vi "Dresden R2R Sputter 03.02.2018 IY24.vi"() -> ()   [LabVIEW 2009] (continued)
        "CH1_2trns_6" <- w28815
        "CH1_2trns_11" <- w28815
        "CH1_2trns_12" <- w28815
        "CH1_2trns_19" <- w28815
        "CH1_2trns_7" <- w28815
        "CH1_2trns_8" <- w28815
      }
    }
    n23486 = case shown="True" "Clean_trnsfr_2_3" {
      frame #0 {
      }
      frame #1 {
        w28814 = i16? 0
        n23487 = local write "Clean_trnsfr_2_3"(w28814) -> ()
        "CH2_3_trns_0" <- w28814
        "CH2_3_trns_1" <- w28814
        "CH2_3_trns_2" <- w28814
        "CH2_3_trns_4" <- w28814
        "CH2_3_trns_7" <- w28814
        "CH2_3_trns_8" <- w28814
        "CH2_3_trns_12" <- w28814
        "CH2_3_trns_15" <- w28814
        "CH2_3_trns_18" <- w28814
        "CH2_3_trns_19" <- w28814
        "CH2_3_trns_11" <- w28814
        "CH2_3_trns_10" <- w28814
        "CH2_3_trns_3" <- w28814
        "CH2_3_trns_5" <- w28814
        "CH2_3_trns_6" <- w28814
        "CH2_3_trns_9" <- w28814
        "CH2_3_trns_14" <- w28814
        "CH2_3_trns_17" <- w28814
        "CH2_3_trns_16" <- w28814
        "CH2_3_trns_13" <- w28814
        "CH2_3_trns_20" <- w28814
      }
    }
    n23488 = case shown="True" "Clean_trnsfr_3_4" {
      frame #0 {
      }
      frame #1 {
        w28813 = i16? 0
        n23489 = local write "Clean_trnsfr_3_4"(w28813) -> ()
        "CH3_4_trns_0" <- w28813
        "CH3_4_trns_1" <- w28813
        "CH3_4_trns_2" <- w28813
        "CH3_4_trns_4" <- w28813
        "CH3_4_trns_7" <- w28813
        "CH3_4_trns_8" <- w28813
        "CH3_4_trns_12" <- w28813
        "CH3_4_trns_15" <- w28813
        "CH3_4_trns_18" <- w28813
        "CH3_4_trns_19" <- w28813
        "CH3_4_trns_10" <- w28813
        "CH3_4_trns_11" <- w28813
        "CH3_4_trns_3" <- w28813
        "CH3_4_trns_5" <- w28813
        "CH3_4_trns_6" <- w28813
        "CH3_4_trns_9" <- w28813
        "CH3_4_trns_14" <- w28813
        "CH3_4_trns_17" <- w28813
        "CH3_4_trns_16" <- w28813
        "CH3_4_trns_13" <- w28813
        "CH3_4_trns_20" <- w28813
      }
    }
    n23490 = case shown="True" "Clean_trnsfr_2_1" {
      frame #0 {
      }
      frame #1 {
        w28812 = i16? 0
        n23491 = local write "Clean_trnsfr_2_1"(w28812) -> ()
        "CH2_1_trns_0" <- w28812
        "CH2_1_trns_1" <- w28812
        "CH2_1_trns_2" <- w28812
        "CH2_1_trns_3" <- w28812
        "CH2_1_trns_4" <- w28812
        "CH2_1_trns_5" <- w28812
        "CH2_1_trns_7" <- w28812
        "CH2_1_trns_6" <- w28812
        "CH2_1_trns_8" <- w28812
        "CH2_1_trns_9" <- w28812
        "CH2_1_trns_10" <- w28812
        "CH2_1_trns_11" <- w28812
        "CH2_1_trns_12" <- w28812
        "CH2_1_trns_14" <- w28812
        "CH2_1_trns_15" <- w28812
        "CH2_1_trns_17" <- w28812
        "CH2_1_trns_18" <- w28812
        "CH2_1_trns_16" <- w28812
        "CH2_1_trns_19" <- w28812
        "CH2_1_trns_13" <- w28812
        "CH2_1_trns_20" <- w28812
      }
    }
    n23492 = case shown="True" "Clean_trnsfr_3_2" {
      frame #0 {
      }
      frame #1 {
        w28811 = i16? 0
        n23493 = local write "Clean_trnsfr_3_2"(w28811) -> ()
        "CH3_2_trns_0" <- w28811
        "CH3_2_trns_1" <- w28811
        "CH3_2_trns_2" <- w28811
        "CH3_2_trns_3" <- w28811
        "CH3_2_trns_4" <- w28811
        "CH3_2_trns_5" <- w28811
        "CH3_2_trns_7" <- w28811
        "CH3_2_trns_6" <- w28811
        "CH3_2_trns_ 8" <- w28811
        "CH3_2_trns_9" <- w28811
        "CH3_2_trns_10" <- w28811
        "CH3_2_trns_11" <- w28811
        "CH3_2_trns_12" <- w28811
        "CH3_2_trns_14" <- w28811
        "CH3_2_trns_15" <- w28811
        "CH3_2_trns_17" <- w28811
        "CH3_2_trns_18" <- w28811
        "CH3_2_trns_16" <- w28811
        "CH3_2_trns_19" <- w28811
        "CH3_2_trns_13" <- w28811
        "CH3_2_trns_20" <- w28811
      }
    }
    n23494 = case shown="True" "Clean_trnsfr_4_3" {
      frame #0 {
      }
      frame #1 {
        w28810 = i16? 0
        n23495 = local write "Clean_trnsfr_4_3"(w28810) -> ()
        "CH4_3_trns_0" <- w28810
        "CH4_3_trns_1" <- w28810
        "CH4_3_trns_2" <- w28810
        "CH4_3_trns_3" <- w28810
        "CH4_3_trns_5" <- w28810
        "CH4_3_trns_7" <- w28810
        "CH4_3_trns_6" <- w28810
        "CH4_3_trns_8" <- w28810
        "CH4_3_trns_9" <- w28810
        "CH4_3_trns_10" <- w28810
        "CH4_3_trns_4" <- w28810
        "CH4_3_trns_11" <- w28810
        "CH4_3_trns_14" <- w28810
        "CH4_3_trns_15" <- w28810
        "CH4_3_trns_17" <- w28810
        "CH4_3_trns_18" <- w28810
        "CH4_3_trns_19" <- w28810
        "CH4_3_trns_16" <- w28810
        "CH4_3_trns_13" <- w28810
        "CH4_3_trns_20" <- w28810
      }
    }
    n23496 = case shown="True" "Routine_check" {
      frame #0 {
      }
      frame #1 {
        w28807 = i16? 0
        n23497 = local write "Routine_check"(w28807) -> ()
        "RC_1" <- w28807
        "RC_2" <- w28807
        "RC_3" <- w28807
        "RC_4" <- w28807
        "RC_5" <- w28807
        "RC_6" <- w28807
        "RC_7" <- w28807
        "RC_8" <- w28807
        "RC_9" <- w28807
        "RC_10" <- w28807
        "RC_11" <- w28807
        "RC_12" <- w28807
        "RC_13" <- w28807
      }
    }
    n23498 = stacked-sequence {
      frame #0 {
        # "MAIN TRANSFER CLEAN"
        n23499 = case shown="True" "Clean_main_trns" {
          frame #0 {
          }
          frame #1 {
            w28809 = i16? 0 ("a1")
            n23500 = local write "Clean_main_trns"(w28809) -> ()
            "MT4" <- w28809
            "MT1" <- w28809
            "MT5" <- w28809
            "MT6" <- w28809
            "MT3" <- w28809
            "MT2" <- w28809
            "MT7" <- w28809
            "MT13" <- w28809
            "MT9" <- w28809
            "MT11" <- w28809
            "MT8" <- w28809
            "MT10" <- w28809
            "MT12" <- w28809
            "MT14" <- w28809
            "MT15" <- w28809
            "MT18" <- w28809
            "MT16" <- w28809
            "MT17" <- w28809
            "MT19" <- w28809
            "MT20" <- w28809
            "MTF" <- w28809
          }
        }
      }
    }
    n23501 = case shown="True" "Clean_MW_Coating" {
      frame #0 {
      }
      frame #1 {
        w28806 = i16? 0 ("a1")
        n23502 = local write "Clean_MW_Coating"(w28806) -> ()
        "SMW1" <- w28806
        "SMW2" <- w28806
        "SMW4" <- w28806
        "SMW5" <- w28806
        "SMW6" <- w28806
        "SMW9" <- w28806
        "SMW8" <- w28806
        "SMW11" <- w28806
        "SMW12" <- w28806
        "SMW13" <- w28806
        "SMW14" <- w28806
        "SMW15" <- w28806
        "SMW3" <- w28806
        "SMW16" <- w28806
        "SMW17" <- w28806
        "SMW18" <- w28806
        "SMW19" <- w28806
        "SMW21" <- w28806
        "SMW22" <- w28806
        "SMW23" <- w28806
        "SMW26" <- w28806
        "SMW7" <- w28806
        "SMW10" <- w28806
        "SMW20" <- w28806
        "SMW18b" <- w28806
        "SMW24" <- w28806
        "SMW25" <- w28806
        "SMW1 2" <- w28806
      }
    }
    n23503 = case shown="True" "Clean_Single_DC1" {
      frame #0 {
      }
      frame #1 {
        w28805 = i16? 0 ("a1")
        n23504 = local write "Clean_Single_DC1"(w28805) -> ()
        "SDC1 1" <- w28805
        "SDC1 2" <- w28805
        "SDC1 3" <- w28805
        "SDC1 4" <- w28805
        "SDC1 5" <- w28805
        "SDC1 6" <- w28805
        "SDC1 7" <- w28805
        "SDC1 8" <- w28805
        "SDC1 9" <- w28805
        "SDC1 10" <- w28805
        "SDC1 11" <- w28805
        "SDC1 13" <- w28805
        "SDC1 14" <- w28805
        "SDC1 17" <- w28805
        "SDC1 18" <- w28805
        "SDC1 20" <- w28805
        "SDC1 21" <- w28805
        "SDC1 22" <- w28805
        "SDC1 23" <- w28805
        "SDC1 24" <- w28805
        "SDC1 25" <- w28805
        "SDC1 26" <- w28805
        "SDC1 27" <- w28805
        "SDC1 28" <- w28805
        "SDC1 29" <- w28805
        "SDC1 30" <- w28805
        "SDC1 21b" <- w28805
        "SDC1 2b" <- w28805
        "SDC1 7b" <- w28805
        "SDC1 10b" <- w28805
        "SDC1 13b" <- w28805
        "SDC1 14b" <- w28805
        "SDC1 27b" <- w28805
        "SDC1 27c" <- w28805
        "SDC1 12" <- w28805
      }
    }
    n23505 = case shown="True" "Clean_Single_DC2" {
      frame #0 {
      }
      frame #1 {
        w28804 = i16? 0 ("a1")
        n23506 = local write "Clean_Single_DC2"(w28804) -> ()
        "SDC2 1" <- w28804
        "SDC2 2" <- w28804
        "SDC2 4" <- w28804
        "SDC2 3" <- w28804
        "SDC2 5" <- w28804
        "SDC2 6" <- w28804
        "SDC2 7" <- w28804
        "SDC2 8" <- w28804
        "SDC2 9" <- w28804
        "SDC2 10" <- w28804
        "SDC2 11" <- w28804
        "SDC2 12" <- w28804
        "SDC2 13" <- w28804
        "SDC2 14" <- w28804
        "SDC2 17" <- w28804
        "SDC2 18" <- w28804
        "SDC2 20" <- w28804
        "SDC2 21" <- w28804
        "SDC2 22" <- w28804
        "SDC2 23" <- w28804
        "SDC2 24" <- w28804
        "SDC2 25" <- w28804
        "SDC2 26" <- w28804
        "SDC2 27" <- w28804
        "SDC2 28" <- w28804
        "SDC2 29" <- w28804
        "SDC2 30" <- w28804
        "SDC2 21b" <- w28804
        "SDC2 3b" <- w28804
        "SDC2 b" <- w28804
        "SDC2 10b" <- w28804
        "SDC2 15" <- w28804
        "SDC2 16" <- w28804
        "SDC2 28b" <- w28804
        "SDC2 28c" <- w28804
        "SDC2 19" <- w28804
      }
    }
    n23507 = case shown="True" "Clean_Single_RF" {
      frame #0 {
      }
      frame #1 {
        w28803 = i16? 0 ("a1")
        n23508 = local write "Clean_Single_RF"(w28803) -> ()
        "SRF 1" <- w28803
        "SRF 2" <- w28803
        "SRF 3" <- w28803
        "SRF 4" <- w28803
        "SRF 5" <- w28803
        "SRF 6" <- w28803
        "SRF 7" <- w28803
        "SRF 8" <- w28803
        "SRF 9" <- w28803
        "SRF 10" <- w28803
        "SRF 11" <- w28803
        "SRF 12" <- w28803
        "SRF 13" <- w28803
        "SRF 14" <- w28803
        "SRF 17" <- w28803
        "SRF 18" <- w28803
        "SRF 19" <- w28803
        "SRF 20" <- w28803
        "SRF 21" <- w28803
        "SRF 22" <- w28803
        "SRF 23" <- w28803
        "SRF 24" <- w28803
        "SRF 25" <- w28803
        "SRF 26" <- w28803
        "SRF 27" <- w28803
        "SRF 28" <- w28803
        "SRF 29" <- w28803
        "SRF 30" <- w28803
        "SRF 21b" <- w28803
        "SRF 4b" <- w28803
        "SRF 7b" <- w28803
        "SRF 8b" <- w28803
        "SRF 27b" <- w28803
        "SRF 27c" <- w28803
        "SRF 15" <- w28803
      }
    }
    n23509 = case shown="True" "Clean_Combo" {
      frame #0 {
      }
      frame #1 {
        w28802 = i16? 0 ("a1")
        n23510 = local write "Clean_Combo"(w28802) -> ()
        "SCMB1" <- w28802
        "SCMB2" <- w28802
        "SCMB3" <- w28802
        "SCMB4" <- w28802
        "SCMB5" <- w28802
        "SCMB6" <- w28802
        "SCMB7" <- w28802
        "SCMB8" <- w28802
        "SCMB9" <- w28802
        "SCMB10" <- w28802
        "SCMB11" <- w28802
        "SCMB12" <- w28802
        "SCMB13" <- w28802
        "SCMB14" <- w28802
        "SCMB15" <- w28802
        "SCMB16" <- w28802
        "SCMB17" <- w28802
        "SCMB18" <- w28802
        "SCMB19" <- w28802
        "SCMB20" <- w28802
        "SCMB21" <- w28802
        "SCMB22" <- w28802
        "SCMB23" <- w28802
        "SCMB24" <- w28802
        "SCMB25" <- w28802
        "SCMB26" <- w28802
        "SCMB27" <- w28802
        "SCMB28" <- w28802
        "SCMB29" <- w28802
        "SCMB30" <- w28802
        "SCMB31" <- w28802
        "SCMB32" <- w28802
        "SCMB33" <- w28802
        "SCMB34" <- w28802
        "SCMB35" <- w28802
        "SCMB36" <- w28802
        "SCMB37" <- w28802
        "SCMB38" <- w28802
        "SCMB39" <- w28802
        "SCMB40" <- w28802
        "SCMB41" <- w28802
        "SCMB42" <- w28802
        "SCMB43" <- w28802
        "SCMB44" <- w28802
        "SCMB45" <- w28802
        "SCMB46" <- w28802
        "SCMB47" <- w28802
        "SCMB48" <- w28802
        "SCMB49" <- w28802
        "SCMB50" <- w28802
        "SCMB51" <- w28802
        "SCMB52" <- w28802
        "SCMB53" <- w28802
        "SCMB54" <- w28802
        "SCMB55" <- w28802
        "SCMB56" <- w28802
        "SCMB57" <- w28802
        "SCMB58" <- w28802
        "SCMB59" <- w28802
        "SCMB60" <- w28802
        "SCMB61" <- w28802
        "SCMB62" <- w28802
        "SCMB63" <- w28802
        "SCMB64" <- w28802
        "SCMB65" <- w28802
        "SCMB66" <- w28802
        "SCMB67" <- w28802
        "SCMB68" <- w28802
        "SCMB69" <- w28802
        "SCMB70" <- w28802
        "SCMB71" <- w28802
        "SCMB72" <- w28802
        "SCMB73" <- w28802
        "SCMB74" <- w28802
        "SCMB75" <- w28802
        "SCMB0" <- w28802
        "SCMB0 2" <- w28802
      }
    }
  }
  n23511 = VISA Close(VISA resource name=w809, error in (no error)=w733) -> ()  [unwired: 1 out]
  n23512 = while {
    stop <- FALSE stop-if-true
    n23513 = local read "Path"() -> (w28838:string)
    n23514 = Wait Until Next ms Multiple(millisecond multiple=u32 300) -> ()  [unwired: 1 out]
    n23515 = String To Path(string=w28838) -> (path=w28839:path)
    n23516 = Not Equal?(x=w28838, y="") -> (x != y?=w28840:bool)
    n23517 = case shown="True" w28840 {
      tunnel: w28839 -> [_ w28936]
      frame #0 {
      }
      frame #1 {
        # "Thickness Monitor AC/DEAC\nMaterial Density\nZ factor\nTooling Factor"
        # "Target Material\nIgnition Power\nTarget clean Power AC/DEAC\nTarget clean Power\nTarget clean Time\nTarget Material\nIgnition Power\nTarget clean Power AC/DEAC\nTarget clean Power\nTarget clean Time\nRegion1 active/deactive\nch2-Coating Power\nch3-Coating Power\nRegion2 active/deactive\nch2-Coating Power\nch3-Coating Power\nRegion3 active/deactive\nch2-Coating Power\nch3-Coating Power\nRegion4 active/deactive\nch2-Coating Power\nch3-Coating Power\nRegion5 active/deactive\nch2-Coating Power\nch3-Coating Power\nInterval Length"
        # "Target Material\nRamp Up Time Active/deactive\nRamp Up Time\nIgnition Power\nTarget Clean  ACT/DEACT\nTarget Clean Power\nTarget Clean Time\nRegion1 active/deactive\nCoating Power\nInterval Length\nRegion2 active/deactive\nCoating Powe\nRegion3 active/deactive\nCoating Power\nRegion4 active/deactive\nCoating Power\nRegion5 active/deactive\nCoating Power\nRamp DownTime activedeactive\nRamp Down Time"
        # "Recipe Selection"
        # "Ar Flow\nSet Pressure"
        # "DC SELECTION\nTarget Material\nIgnition Power\nTarget Clean  ACT/DEACT\nTarget Clean Power\nTarget Clean Time\nRegion1 active/deactive\nCoating Power\nInterval Length\nRegion2 active/deactive\nCoating Powe\nRegion3 active/deactive\nCoating Power\nRegion4 active/deactive\nCoating Power\nRegion5 active/deactive\nCoating Power"
        # "Microwave Plasma Power\n\nMicrowave Duration\nMicrowave Times"
        # "Coating Selection"
        # "Thickness Selection\nTarget Thickness Value\nTime"
        # "Min. Diameter\nMax. Diameter\nWeb Thickness\nWeb Speed\nTension  Value\nTotal Length"
        # "Web Selection"
        # "Substrate Material"
        # "Recipe Name"
        n23518 = call-poly <vilib>:"Read From Spreadsheet File.vi"("file path (dialog if empty)"=w28936) -> ("all rows"=w29282:string[][])  [unwired: 6 in, 4 out]
        n23519 = Index Array(array=w29282, index (row) #1=1 ("disabled index (row)"), index (col) #1=3 ("disabled index (col)"), index (row) #2=4 ("disabled index (row)"), index (col) #2=2 ("disabled index (col)"), index (row) #3=7 ("disabled index (row)"), index (col) #3=2 ("disabled index (col)"), index (row) #4=9 ("disabled index (row)"), index (col) #4=3 ("disabled index (col)"), index (row) #5=12 ("disabled index (row)"), index (col) #5=2 ("disabled index (col)"), index (row) #6=13 ("disabled index (row)"), index (col) #6=2 ("disabled index (col)"), index (row) #7=14 ("disabled index (row)"), index (col) #7=2 ("disabled index (col)"), index (row) #8=15 ("disabled index (row)"), index (col) #8=2 ("disabled index (col)"), index (row) #9=16 ("disabled index (row)"), index (col) #9=2 ("disabled index (col)"), index (row) #10=17 ("disabled index (row)"), index (col) #10=3 ("disabled index (col)"), index (row) #11=20 ("disabled index (row)"), index (col) #11=2 ("disabled index (col)"), index (row) #12=21 ("disabled index (row)"), index (col) #12=3 ("disabled index (col)"), index (row) #13=22 ("disabled index (row)"), index (col) #13=3 ("disabled index (col)"), index (row) #14=25 ("disabled index (row)"), index (col) #14=2 ("disabled index (col)"), index (row) #15=27 ("disabled index (row)"), index (col) #15=1 ("disabled index (col)"), index (row) #16=28 ("disabled index (row)"), index (col) #16=1 ("disabled index (col)"), index (row) #17=29 ("disabled index (row)"), index (col) #17=4 ("disabled index (col)"), index (row) #18=34 ("disabled index (row)"), index (col) #18=2 ("disabled index (col)"), index (row) #19=35 ("disabled index (row)"), index (col) #19=2 ("disabled index (col)"), index (row) #20=36 ("disabled index (row)"), index (col) #20=2 ("disabled index (col)"), index (row) #21=37 ("disabled index (row)"), index (col) #21=2 ("disabled index (col)"), index (row) #22=38 ("disabled index (row)"), index (col) #22=2 ("disabled index (col)"), index (row) #23=39 ("disabled index (row)"), index (col) #23=2 ("disabled index (col)"), index (row) #24=40 ("disabled index (row)"), index (col) #24=3 ("disabled index (col)"), index (row) #25=41 ("disabled index (row)"), index (col) #25=2 ("disabled index (col)"), index (row) #26=42 ("disabled index (row)"), index (col) #26=2 ("disabled index (col)"), index (row) #27=43 ("disabled index (row)"), index (col) #27=3 ("disabled index (col)"), index (row) #28=44 ("disabled index (row)"), index (col) #28=2 ("disabled index (col)"), index (row) #29=45 ("disabled index (row)"), index (col) #29=3 ("disabled index (col)"), index (row) #30=46 ("disabled index (row)"), index (col) #30=2 ("disabled index (col)"), index (row) #31=47 ("disabled index (row)"), index (col) #31=3 ("disabled index (col)"), index (row) #32=48 ("disabled index (row)"), index (col) #32=2 ("disabled index (col)"), index (row) #33=49 ("disabled index (row)"), index (col) #33=3 ("disabled index (col)"), index (row) #34=50 ("disabled index (row)"), index (col) #34=2 ("disabled index (col)"), index (row) #35=53 ("disabled index (row)"), index (col) #35=2 ("disabled index (col)"), index (row) #36=54 ("disabled index (row)"), index (col) #36=2 ("disabled index (col)"), index (row) #37=55 ("disabled index (row)"), index (col) #37=2 ("disabled index (col)"), index (row) #38=56 ("disabled index (row)"), index (col) #38=2 ("disabled index (col)"), index (row) #39=57 ("disabled index (row)"), index (col) #39=2 ("index (col)"), index (row) #40=58 ("disabled index (row)"), index (col) #40=2 ("index (col)"), index (row) #41=59 ("disabled index (row)"), index (col) #41=2 ("index (col)"), index (row) #42=60 ("disabled index (row)"), index (col) #42=3 ("index (col)"), index (row) #43=61 ("disabled index (row)"), index (col) #43=2 ("index (col)"), index (row) #44=62 ("disabled index (row)"), index (col) #44=2 ("index (col)"), index (row) #45=63 ("disabled index (row)"), index (col) #45=3 ("index (col)"), index (row) #46=64 ("disabled index (row)"), index (col) #46=2 ("index (col)"), index (row) #47=65 ("disabled index (row)"), index (col) #47=3 ("disabled index (row)"), index (row) #48=66 ("disabled index (row)"), index (col) #48=2 ("disabled index (col)"), index (row) #49=67 ("disabled index (row)"), index (col) #49=3 ("index (col)"), index (row) #50=68 ("disabled index (row)"), index (col) #50=2 ("index (col)"), index (row) #51=69 ("disabled index (row)"), index (col) #51=3 ("index (col)"), index (row) #52=70 ("disabled index (row)"), index (col) #52=2 ("index (col)"), index (row) #53=71 ("disabled index (row)"), index (col) #53=2 ("disabled index (col)"), index (row) #54=72 ("disabled index (row)"), index (col) #54=3 ("index (col)"), index (row) #55=78 ("disabled index (row)"), index (col) #55=2 ("index (col)"), index (row) #56=79 ("disabled index (row)"), index (col) #56=2 ("index (col)"), index (row) #57=80 ("disabled index (row)"), index (col) #57=2 ("index (col)"), index (row) #58=81 ("disabled index (row)"), index (col) #58=2 ("index (col)"), index (row) #59=82 ("disabled index (row)"), index (col) #59=2 ("index (col)"), index (row) #60=83 ("disabled index (row)"), index (col) #60=2 ("index (col)"), index (row) #61=84 ("disabled index (row)"), index (col) #61=2 ("index (col)"), index (row) #62=85 ("disabled index (row)"), index (col) #62=2 ("index (col)"), index (row) #63=86 ("disabled index (row)"), index (col) #63=2 ("index (col)"), index (row) #64=87 ("disabled index (row)"), index (col) #64=2 ("index (col)"), index (row) #65=88 ("disabled index (row)"), index (col) #65=3 ("index (col)"), index (row) #66=89 ("disabled index (row)"), index (col) #66=2 ("index (col)"), index (row) #67=90 ("disabled index (row)"), index (col) #67=2 ("index (col)"), index (row) #68=91 ("disabled index (row)"), index (col) #68=3 ("index (col)"), index (row) #69=92 ("disabled index (row)"), index (col) #69=2 ("index (col)"), index (row) #70=93 ("disabled index (row)"), index (col) #70=2 ("index (col)"), index (row) #71=94 ("disabled index (row)"), index (col) #71=3 ("index (col)"), index (row) #72=95 ("disabled index (row)"), index (col) #72=2 ("disabled index (col)"), index (row) #73=96 ("disabled index (row)"), index (col) #73=2 ("index (col)"), index (row) #74=97 ("disabled index (row)"), index (col) #74=3 ("index (col)"), index (row) #75=98 ("disabled index (row)"), index (col) #75=2 ("index (col)"), index (row) #76=99 ("disabled index (row)"), index (col) #76=2 ("index (col)"), index (row) #77=100 ("disabled index (row)"), index (col) #77=3 ("index (col)"), index (row) #78=101 ("disabled index (row)"), index (col) #78=2 ("index (col)"), index (row) #79=102 ("disabled index (row)"), index (col) #79=2 ("index (col)"), index (row) #80=103 ("disabled index (row)"), index (col) #80=2 ("index (col)"), index (row) #81=104 ("disabled index (row)"), index (col) #81=2 ("disabled index (row)"), index (row) #82=108 ("disabled index (row)"), index (col) #82=2 ("index (col)"), index (row) #83=109 ("disabled index (row)"), index (col) #83=2 ("index (col)"), index (row) #84=113 ("disabled index (row)"), index (col) #84=2 ("index (col)"), index (row) #85=114 ("disabled index (row)"), index (col) #85=3 ("index (col)"), index (row) #86=115 ("disabled index (row)"), index (col) #86=2 ("index (col)"), index (row) #87=116 ("disabled index (row)"), index (col) #87=2 ("index (col)")) -> (element #1=w29273:string, element #2=w29269:string, element #3=w29268:string, element #4=w29266:string, element #5=w29257:string, element #6=w29256:string, element #7=w29255:string, element #8=w29252:string, element #9=w29249:string, element #10=w29248:string, element #11=w29247:string, element #12=w29242:string, element #13=w29241:string, element #14=w29239:string, element #15=w29236:string, element #16=w28926:string, element #17=w28925:string, element #18=w28924:string, element #19=w29185:string, element #20=w29184:string, element #21=w29183:string, element #22=w29182:string, element #23=w29181:string, element #24=w29180:string, element #25=w29179:string, element #26=w29178:string, element #27=w29177:string, element #28=w29176:string, element #29=w29175:string, element #30=w29174:string, element #31=w29173:string, element #32=w29172:string, element #33=w29171:string, element #34=w29168:string, element #35=w29133:string, element #36=w29130:string, element #37=w29128:string, element #38=w29097:string, element #39=w29096:string, element #40=w29095:string, element #41=w29094:string, element #42=w29093:string, element #43=w29092:string, element #44=w29091:string, element #45=w29090:string, element #46=w29089:string, element #47=w29088:string, element #48=w29087:string, element #49=w29086:string, element #50=w29085:string, element #51=w29084:string, element #52=w29083:string, element #53=w29082:string, element #54=w29081:string, element #55=w29021:string, element #56=w29020:string, element #57=w29019:string, element #58=w28998:string, element #59=w28997:string, element #60=w28996:string, element #61=w28995:string, element #62=w28994:string, element #63=w28992:string, element #64=w28979:string, element #65=w28978:string, element #66=w28977:string, element #67=w28976:string, element #68=w28971:string, element #69=w28970:string, element #70=w28969:string, element #71=w28968:string, element #72=w28965:string, element #73=w28964:string, element #74=w28963:string, element #75=w28962:string, element #76=w28959:string, element #77=w28958:string, element #78=w28956:string, element #79=w28955:string, element #80=w28954:string, element #81=w28913:string, element #82=w28912:string, element #83=w28906:string, element #84=w28904:string, element #85=w28903:string, element #86=w28902:string, element #87=w28901:string)
        n23520 = Equal?(x="Active", y=w28904) -> (x = y?=w28905:bool)
        n23521 = case shown="True" w28905 {
          frame #0 {
            n23522 = local write "Thickness_Monitor_Active"(FALSE ("Thickness_Monitor_Active")) -> ()
          }
          frame #1 {
            n23523 = local write "Thickness_Monitor_Active"(TRUE ("Thickness_Monitor_Active")) -> ()
          }
        }
        n23524 = Scan Value(string=w28913, format string="") -> (value=w28915:dbl)  [unwired: 1 in, 1 out]
        n23525 = Scan Value(string=w28912, format string="") -> (value=w28950:dbl)  [unwired: 1 in, 1 out]
        n23526 = Scan Value(string=w28906, format string="") -> (value=w28947:dbl)  [unwired: 1 in, 1 out]
        n23527 = Scan Value(string=w28903, format string="") -> (value=w28945:dbl)  [unwired: 1 in, 1 out]
        n23528 = Scan Value(string=w28902, format string="") -> (value=w28942:dbl)  [unwired: 1 in, 1 out]
        n23529 = Scan Value(string=w28901, format string="") -> (value=w28941:dbl)  [unwired: 1 in, 1 out]
        n23530 = local write "R Material_density"(w28945) -> ()
        n23531 = local write "R Z_factor"(w28942) -> ()
        n23532 = local write "R Toooling_factor"(w28941) -> ()
        n23533 = local write "R Cmb Number of pairs"(w28915) -> ()
        n23534 = local write "R Argon Flow sccm"(w28950) -> ()
        n23535 = local write "R Set Pressure mtorr"(w28947) -> ()
        n23536 = local write "Recipe Name"(w29273) -> ()
        n23537 = local write "Substrate Material"(w29269) -> ()
        n23538 = local write "R Cmb Ch3 Target material"(w28996) -> ()
        n23539 = local write "R Cmb Ch2 Target material"(w29021) -> ()
        n23540 = Scan Value(string=w28998, format string="") -> (value=w29016:dbl)  [unwired: 1 in, 1 out]
        n23541 = Scan Value(string=w29020, format string="") -> (value=w29024:dbl)  [unwired: 1 in, 1 out]
        n23542 = Scan Value(string=w28997, format string="") -> (value=w29015:dbl)  [unwired: 1 in, 1 out]
        n23543 = Scan Value(string=w28995, format string="") -> (value=w29013:dbl)  [unwired: 1 in, 1 out]
        n23544 = Scan Value(string=w28979, format string="") -> (value=w29009:dbl)  [unwired: 1 in, 1 out]
        n23545 = Scan Value(string=w28992, format string="") -> (value=w29010:dbl)  [unwired: 1 in, 1 out]
        n23546 = Scan Value(string=w28970, format string="") -> (value=w28973:dbl)  [unwired: 1 in, 1 out]
        n23547 = Scan Value(string=w28964, format string="") -> (value=w28966:dbl)  [unwired: 1 in, 1 out]
        n23548 = Scan Value(string=w28969, format string="") -> (value=w28972:dbl)  [unwired: 1 in, 1 out]
        n23549 = Scan Value(string=w28955, format string="") -> (value=w28953:dbl)  [unwired: 1 in, 1 out]
        n23550 = Scan Value(string=w28976, format string="") -> (value=w28974:dbl)  [unwired: 1 in, 1 out]
        n23551 = Scan Value(string=w28965, format string="") -> (value=w28967:dbl)  [unwired: 1 in, 1 out]
        n23552 = Scan Value(string=w28977, format string="") -> (value=w28975:dbl)  [unwired: 1 in, 1 out]
        n23553 = Scan Value(string=w28956, format string="") -> (value=w28957:dbl)  [unwired: 1 in, 1 out]
        n23554 = Scan Value(string=w28954, format string="") -> (value=w28952:dbl)  [unwired: 1 in, 1 out]
        n23555 = local write "R Cmb Ch2 DC Ignition Power"(w29024) -> ()
        n23556 = Scan Value(string=w28962, format string="") -> (value=w28961:dbl)  [unwired: 1 in, 1 out]
        n23557 = Scan Value(string=w28959, format string="") -> (value=w28960:dbl)  [unwired: 1 in, 1 out]
        n23558 = local write "R Cmb Ch2 DC Target Clean Power"(w29016) -> ()
        n23559 = local write "R Cmb Ch2 DC Target Clean Time"(w29015) -> ()
        n23560 = Equal?(x="Active", y=w28971) -> (x = y?=w29005:bool)
        n23561 = Equal?(x="Active", y=w28978) -> (x = y?=w29007:bool)
        n23562 = local write "R Cmb Ch3 DC Ignition Power"(w29013) -> ()
        n23563 = local write "R Cmb Ch3 DC Target Clean Power"(w29010) -> ()
        n23564 = local write "R Cmb Ch3 DC Target Clean Time"(w29009) -> ()
        n23565 = Equal?(x="Active", y=w28968) -> (x = y?=w29003:bool)
        n23566 = Equal?(x="Active", y=w29019) -> (x = y?=w29022:bool)
        n23567 = Equal?(x="Active", y=w28994) -> (x = y?=w29011:bool)
        n23568 = local write "R Cmb Ch2 Step1 Coating Power"(w28975) -> ()
        n23569 = local write "R Cmb Ch3 Step1 Coating Power"(w28974) -> ()
        n23570 = Equal?(x="Active", y=w28963) -> (x = y?=w29000:bool)
        n23571 = case shown="False" w29005 {
          frame #0 {
            n23572 = local write "R Cmb Ch2 Step2 Coating Power Active"(FALSE ("R Cmb Ch2 Step2 Coating Power Active")) -> ()
          }
          frame #1 {
            n23573 = local write "R Cmb Ch2 Step2 Coating Power Active"(TRUE ("R Cmb Ch2 Step2 Coating Power Active")) -> ()
          }
        }
        n23574 = local write "R Cmb Ch3 Step5 Coating Power"(w28953) -> ()
        n23575 = Equal?(x="Single", y=w29268) -> (x = y?=w29279:bool)
        n23576 = case shown="False" w29007 {
          frame #0 {
            n23577 = local write "R Cmb Ch2 Step1 Coating Power Active"(FALSE ("R Cmb Ch2 Step1 Coating Power Active")) -> ()
          }
          frame #1 {
            n23578 = local write "R Cmb Ch2 Step1 Coating Power Active"(TRUE ("R Cmb Ch2 Step1 Coating Power Active")) -> ()
          }
        }
        n23579 = case shown="False" w29022 {
          frame #0 {
            n23580 = local write "R Cmb Ch2 DC Target Clean Power Active"(FALSE ("R Cmb Ch2 DC Target Clean Power Active")) -> ()
          }
          frame #1 {
            n23581 = local write "R Cmb Ch2 DC Target Clean Power Active"(TRUE ("R Cmb Ch2 DC Target Clean Power Active")) -> ()
          }
        }
        n23582 = case shown="False" w29003 {
          frame #0 {
            n23583 = local write "R Cmb Ch2 Step3 Coating Power Active"(FALSE ("R Cmb Ch2 Step3 Coating Power Active")) -> ()
          }
          frame #1 {
            n23584 = local write "R Cmb Ch2 Step3 Coating Power Active"(TRUE ("R Cmb Ch2 Step3 Coating Power Active")) -> ()
          }
        }
        n23585 = Equal?(x="Active", y=w28958) -> (x = y?=w28999:bool)
        n23586 = local write "R Cmb Interval length"(w28952) -> ()
        n23587 = Equal?(x="Web", y=w29266) -> (x = y?=w29350:bool)
        n23588 = local write "R Cmb Ch2 Step5 Coating Power"(w28957) -> ()
        n23589 = case shown="False" w29011 {
          frame #0 {
            n23590 = local write "R Cmb Ch3 DC Target Clean Power Active"(FALSE ("R Cmb Ch3 DC Target Clean Power Active")) -> ()
          }
          frame #1 {
            n23591 = local write "R Cmb Ch3 DC Target Clean Power Active"(TRUE ("R Cmb Ch3 DC Target Clean Power Active")) -> ()
          }
        }
        n23592 = local write "R Cmb Ch2 Step3 Coating Power"(w28967) -> ()
        n23593 = local write "R Cmb Ch2 Step4 Coating Power"(w28961) -> ()
        n23594 = local write "R Cmb Ch3 Step3 Coating Power"(w28966) -> ()
        n23595 = local write "R Cmb Ch3 Step4 Coating Power"(w28960) -> ()
        n23596 = case shown="True" w29000 {
          frame #0 {
            n23597 = local write "R Cmb Ch2 Step4 Coating Power Active"(FALSE ("R Cmb Ch2 Step4 Coating Power Active")) -> ()
          }
          frame #1 {
            n23598 = local write "R Cmb Ch2 Step4 Coating Power Active"(TRUE ("R Cmb Ch2 Step4 Coating Power Active")) -> ()
          }
        }
        n23599 = Equal?(x="Combination", y=w29268) -> (x = y?=w29280:bool)
        n23600 = local write "R Cmb Ch2 Step2 Coating Power"(w28973) -> ()
        n23601 = local write "R Cmb Ch3 Step2 Coating Power"(w28972) -> ()
        n23602 = Equal?(x="Other", y=w29266) -> (x = y?=w29349:bool)
        n23603 = case shown="True" w28999 {
          frame #0 {
            n23604 = local write "R Cmb Ch2 Step5 Coating Power Active"(FALSE ("R Cmb Ch2 Step5 Coating Power Active")) -> ()
          }
          frame #1 {
            n23605 = local write "R Cmb Ch2 Step5 Coating Power Active"(TRUE ("R Cmb Ch2 Step5 Coating Power Active")) -> ()
          }
        }
        n23606 = local write "R Single DC Target material"(w29185) -> ()
        n23607 = Equal?(x="DC Sputter", y=w29239) -> (x = y?=w29291:bool)
        n23608 = Equal?(x="Microwave Plasma", y=w29239) -> (x = y?=w29292:bool)
        n23609 = Equal?(x="RF Sputter", y=w29239) -> (x = y?=w29287:bool)
        n23610 = Equal?(x="Thickness", y=w29247) -> (x = y?=w29306:bool)
        n23611 = Build Array(FALSE, w29279, w29280) -> (w29275:bool[])
        n23612 = Equal?(x="Active", y=w29183) -> (x = y?=w29212:bool)
        n23613 = Equal?(x="Active", y=w29180) -> (x = y?=w29207:bool)
        n23614 = Build Array(FALSE, w29350, w29349) -> (w29354:bool[])
        n23615 = Equal?(x="Time", y=w29247) -> (x = y?=w29307:bool)
        n23616 = Equal?(x="Active", y=w29177) -> (x = y?=w29206:bool)
        n23617 = Scan Value(string=w29184, format string="") -> (value=w29214:dbl)  [unwired: 1 in, 1 out]
        n23618 = Equal?(x="Active", y=w29175) -> (x = y?=w29203:bool)
        n23619 = local write "R Single RF Target material"(w29133) -> ()
        n23620 = Boolean Array To Number(Boolean array=w29275) -> (number=w29276:u32)
        n23621 = Equal?(x="Active", y=w29173) -> (x = y?=w29202:bool)
        n23622 = Equal?(x="Active", y=w29171) -> (x = y?=w29187:bool)
        n23623 = case shown="True" w29212 {
          frame #0 {
            n23624 = local write "R Single DC Target Clean"(FALSE ("R Single DC Target Clean")) -> ()
          }
          frame #1 {
            n23625 = local write "R Single DC Target Clean"(TRUE ("R Single DC Target Clean")) -> ()
          }
        }
        n23626 = Boolean Array To Number(Boolean array=w29354) -> (number=w29353:u32)
        n23627 = case shown="True" w29207 {
          frame #0 {
            n23628 = local write "R Single DC Step1 Coating Power Active"(FALSE ("R Single DC Step1 Coating Power Active")) -> ()
          }
          frame #1 {
            n23629 = local write "R Single DC Step1 Coating Power Active"(TRUE ("R Single DC Step1 Coating Power Active")) -> ()
          }
        }
        n23630 = Scan Value(string=w29182, format string="") -> (value=w29196:dbl)  [unwired: 1 in, 1 out]
        n23631 = Scan Value(string=w29181, format string="") -> (value=w29195:dbl)  [unwired: 1 in, 1 out]
        n23632 = Equal?(x="Active", y=w29130) -> (x = y?=w29166:bool)
        n23633 = Scan Value(string=w29179, format string="") -> (value=w29210:dbl)  [unwired: 1 in, 1 out]
        n23634 = Mantissa & Exponent(0:w29276) -> (2:w29281:dbl)  [unwired: 1 out]
        n23635 = Equal?(x="Active", y=w29093) -> (x = y?=w29163:bool)
        n23636 = Equal?(x="Active", y=w29096) -> (x = y?=w29199:bool)
        n23637 = Equal?(x="Active", y=w29090) -> (x = y?=w29160:bool)
        n23638 = Equal?(x="Active", y=w29088) -> (x = y?=w29159:bool)
        n23639 = Scan Value(string=w29178, format string="") -> (value=w29194:dbl)  [unwired: 1 in, 1 out]
        n23640 = Equal?(x="Active", y=w29086) -> (x = y?=w29156:bool)
        n23641 = case shown="False" w29206 {
          frame #0 {
            n23642 = local write "R Single DC Step2 Coating Power Active"(FALSE ("R Single DC Step2 Coating Power Active")) -> ()
          }
          frame #1 {
            n23643 = local write "R Single DC Step2 Coating Power Active"(TRUE ("R Single DC Step2 Coating Power Active")) -> ()
          }
        }
        n23644 = local write "R Single DC Ignition Power"(w29214) -> ()
        n23645 = case shown="False" w29203 {
          frame #0 {
            n23646 = local write "R Single DC Step3 Coating Power Active"(FALSE ("R Single DC Step3 Coating Power Active")) -> ()
          }
          frame #1 {
            n23647 = local write "R Single DC Step3 Coating Power Active"(TRUE ("R Single DC Step3 Coating Power Active")) -> ()
          }
        }
        n23648 = Scan Value(string=w29097, format string="") -> (value=w29125:dbl)  [unwired: 1 in, 1 out]
        n23649 = Equal?(x="Active", y=w29084) -> (x = y?=w29140:bool)
        n23650 = Mantissa & Exponent(0:w29353) -> (2:w29348:dbl)  [unwired: 1 out]
        n23651 = Build Array(FALSE, w29306, w29307) -> (w29302:bool[])
        n23652 = Scan Value(string=w29176, format string="") -> (value=w29191:dbl)  [unwired: 1 in, 1 out]
        n23653 = case shown="False" w29202 {
          frame #0 {
            n23654 = local write "R Single DC Step4 Coating Power Active"(FALSE ("R Single DC Step4 Coating Power Active")) -> ()
          }
          frame #1 {
            n23655 = local write "R Single DC Step4 Coating Power Active"(TRUE ("R Single DC Step4 Coating Power Active")) -> ()
          }
        }
        n23656 = Scan Value(string=w29168, format string="") -> (value=w29170:dbl)  [unwired: 1 in, 1 out]
        n23657 = case shown="True" w29187 {
          frame #0 {
            n23658 = local write "R Single DC Step5 Coating Power Active"(FALSE ("R Single DC Step5 Coating Power Active")) -> ()
          }
          frame #1 {
            n23659 = local write "R Single DC Step5 Coating Power Active"(TRUE ("R Single DC Step5 Coating Power Active")) -> ()
          }
        }
        n23660 = Scan Value(string=w29172, format string="") -> (value=w29188:dbl)  [unwired: 1 in, 1 out]
        n23661 = Scan Value(string=w29174, format string="") -> (value=w29190:dbl)  [unwired: 1 in, 1 out]
        n23662 = Equal?(x="Active", y=w29082) -> (x = y?=w29135:bool)
        n23663 = Scan Value(string=w29128, format string="") -> (value=w29164:dbl)  [unwired: 1 in, 1 out]
        n23664 = Scan Value(string=w29091, format string="") -> (value=w29148:dbl)  [unwired: 1 in, 1 out]
        n23665 = Scan Value(string=w29092, format string="") -> (value=w29154:dbl)  [unwired: 1 in, 1 out]
        n23666 = Scan Value(string=w29257, format string="") -> (value=w29262:dbl)  [unwired: 1 in, 1 out]
        n23667 = Scan Value(string=w29256, format string="") -> (value=w29261:dbl)  [unwired: 1 in, 1 out]
        n23668 = Scan Value(string=w29242, format string="") -> (value=w29244:dbl)  [unwired: 1 in, 1 out]
        n23669 = Scan Value(string=w29241, format string="") -> (value=w29243:dbl)  [unwired: 1 in, 1 out]
        n23670 = Scan Value(string=w29255, format string="") -> (value=w29260:dbl)  [unwired: 1 in, 1 out]
        n23671 = Scan Value(string=w29252, format string="") -> (value=w29259:dbl)  [unwired: 1 in, 1 out]
        n23672 = Scan Value(string=w29249, format string="") -> (value=w29258:dbl)  [unwired: 1 in, 1 out]
        n23673 = Scan Value(string=w29248, format string="") -> (value=w28935:dbl)  [unwired: 1 in, 1 out]
        n23674 = Scan Value(string=w29094, format string="") -> (value=w29150:dbl)  [unwired: 1 in, 1 out]
        n23675 = Scan Value(string=w29095, format string="") -> (value=w29152:dbl)  [unwired: 1 in, 1 out]
        n23676 = case shown="True" w29166 {
          frame #0 {
            n23677 = local write "R Single RF Ramp up"(FALSE ("R Single RF Ramp up")) -> ()
          }
          frame #1 {
            n23678 = local write "R Single RF Ramp up"(TRUE ("R Single RF Ramp up")) -> ()
          }
        }
        n23679 = Scan Value(string=w29089, format string="") -> (value=w29146:dbl)  [unwired: 1 in, 1 out]
        n23680 = local write "R Single DC Step1 Coating Power"(w29210) -> ()
        n23681 = case shown="False" w29199 {
          frame #0 {
            n23682 = local write "R Single RF Target Clean"(FALSE ("R Single RF Target Clean")) -> ()
          }
          frame #1 {
            n23683 = local write "R Single RF Target Clean"(TRUE ("R Single RF Target Clean")) -> ()
          }
        }
        n23684 = case shown="False" w29163 {
          frame #0 {
            n23685 = local write "R Single RF Step1 Coating Power Active"(FALSE ("R Single RF Step1 Coating Power Active")) -> ()
          }
          frame #1 {
            n23686 = local write "R Single RF Step1 Coating Power Active"(TRUE ("R Single RF Step1 Coating Power Active")) -> ()
          }
        }
        n23687 = case shown="False" w29160 {
          frame #0 {
            n23688 = local write "R Single RF Step2 Coating Power Active"(FALSE ("R Single RF Step2 Coating Power Active")) -> ()
          }
          frame #1 {
            n23689 = local write "R Single RF Step2 Coating Power Active"(TRUE ("R Single RF Step2 Coating Power Active")) -> ()
          }
        }
        n23690 = case shown="False" w29159 {
          frame #0 {
            n23691 = local write "R Single RF Step3 Coating Power Active"(FALSE ("R Single RF Step3 Coating Power Active")) -> ()
          }
          frame #1 {
            n23692 = local write "R Single RF Step3 Coating Power Active"(TRUE ("R Single RF Step3 Coating Power Active")) -> ()
          }
        }
        n23693 = case shown="False" w29156 {
          frame #0 {
            n23694 = local write "R Single RF Step4 Coating Power Active"(FALSE ("R Single RF Step4 Coating Power Active")) -> ()
          }
          frame #1 {
            n23695 = local write "R Single RF Step4 Coating Power Active"(TRUE ("R Single RF Step4 Coating Power Active")) -> ()
          }
        }
        n23696 = local write "R Single DC Interval length"(w29194) -> ()
        n23697 = Scan Value(string=w29087, format string="") -> (value=w29144:dbl)  [unwired: 1 in, 1 out]
        n23698 = Scan Value(string=w29236, format string="") -> (value=w28900:dbl)  [unwired: 1 in, 1 out]
        n23699 = case shown="False" w29140 {
          frame #0 {
            n23700 = local write "R Single RF Step5 Coating Power Active"(FALSE ("R Single RF Step5 Coating Power Active")) -> ()
          }
          frame #1 {
            n23701 = local write "R Single RF Step5 Coating Power Active"(TRUE ("R Single RF Step5 Coating Power Active")) -> ()
          }
        }
        n23702 = Boolean Array To Number(Boolean array=w29302) -> (number=w29303:u32)
        n23703 = Scan Value(string=w28925, format string="") -> (value=w29234:dbl)  [unwired: 1 in, 1 out]
        n23704 = case shown="False" w29135 {
          frame #0 {
            n23705 = local write "R Single RF Ramp down"(FALSE ("R Single RF Ramp down")) -> ()
          }
          frame #1 {
            n23706 = local write "R Single RF Ramp down"(TRUE ("R Single RF Ramp down")) -> ()
          }
        }
        n23707 = Scan Value(string=w29085, format string="") -> (value=w29142:dbl)  [unwired: 1 in, 1 out]
        n23708 = Scan Value(string=w29081, format string="") -> (value=w29134:dbl)  [unwired: 1 in, 1 out]
        n23709 = Scan Value(string=w28926, format string="") -> (value=w29233:dbl)  [unwired: 1 in, 1 out]
        n23710 = Scan Value(string=w29083, format string="") -> (value=w29138:dbl)  [unwired: 1 in, 1 out]
        n23711 = local write "R Single DC Target Clean Power"(w29196) -> ()
        n23712 = local write "R Single DC Step2 Coating Power"(w29191) -> ()
        n23713 = local write "R Single DC Step3 Coating Power"(w29190) -> ()
        n23714 = local write "R Single RF Ramp up Time"(w29164) -> ()
        n23715 = Build Array(FALSE, w29292, w29291, w29287) -> (w29296:bool[])
        n23716 = local write "R_Duration"(w29243) -> ()
        n23717 = local write "R Single DC Target Clean Time"(w29195) -> ()
        n23718 = local write "R Single RF Ignition Power"(w29125) -> ()
        n23719 = Equal?(x="Chamber II", y=w28924) -> (x = y?=w28934:bool)
        n23720 = local write "R Single RF Target Clean Time"(w29150) -> ()
        n23721 = local write "R Single RF  Step1 Coating Power"(w29154) -> ()
        n23722 = local write "R Single RF Target Clean Power"(w29152) -> ()
        n23723 = Mantissa & Exponent(0:w29303) -> (2:w29300:dbl)  [unwired: 1 out]
        n23724 = local write "R Single DC Step5 Coating Power"(w29170) -> ()
        n23725 = Equal?(x=w28924, y="Chamber III") -> (x = y?=w28927:bool)
        n23726 = local write "R_Target Thickness Value"(w29244) -> ()